vi "pharmaBot_v0.019.vi"() -> ()   [LabVIEW 2015] (continued)
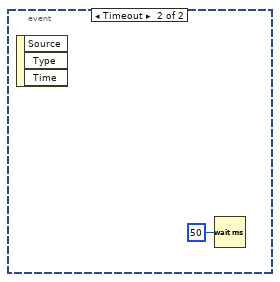
[diagram p2: hidden frame]
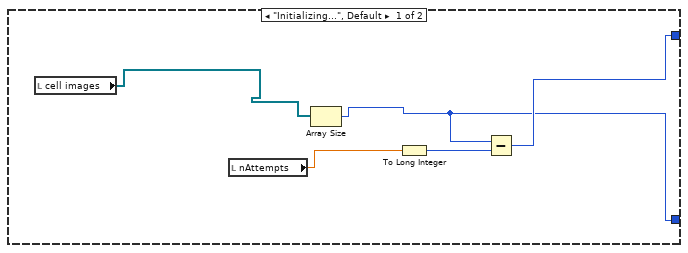
[diagram p4: hidden frame]
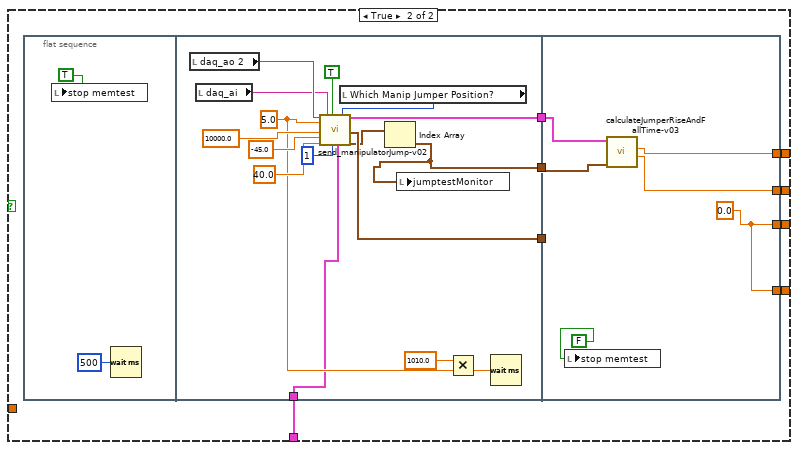
[diagram p14: hidden frame]
              }
              frame "manipulator 2" {
                n1843 = Unbundle By Name(w2697) -> ("manip 2"=w2696:refnum<vi>)
              }
              frame "manipulator 3" {
                n1844 = Unbundle By Name(w2699) -> ("manip 3"=w2698:refnum<vi>)
              }
              frame "manipulator 4" {
                n1845 = Unbundle By Name(w2701) -> ("manip 4"=w2700:refnum<vi>)
              }
            }
            n1846 = property class="Clust (strict)"(reference=w2692) -> (error out=w2689:errorcluster, "Value"=w2691:T25)  [unwired: 1 in, 1 out]
            n1847 = Unbundle By Name(w2691) -> ("actuator"=w2687:T26, "gamma (deg)"=w2678:dbl)
            n1848 = expression code="(x/180.0)*pi" "degrees to radians"(w2678) -> (w2677:dbl)
            n1849 = Unbundle By Name(w2687) -> ("Actuator COM"=w2684:refnum<visa-resource-name>)  [unwired: 1 out]
            n1850 = Sine(x=w2677) -> (sin(x)=w2675:dbl)
            n1851 = Cosine(x=w2677) -> (cos(x)=w2676:dbl)
            n1852 = call "sc_adjustMotion.vi"("error in (no error)"=w2689, "motion"=scope_motion."fast", "VISA handle"=w2684) -> ("error out"=w2688:errorcluster)  [unwired: 7 in, 1 out]
            n1853 = Multiply(x=w2674, y=w2676) -> (x*y=w2672:dbl)
            n1854 = Multiply(x=w2674, y=w2675) -> (x*y=w2673:dbl)
            n1855 = Build Array(w2672, 0, w2673) -> (w2682:dbl[])
            n1856 = call "move manipulator abs xyz.vi"("blocking?"=TRUE, "which manipulator"=w2683, "error in (no error)"=w2688, "transform cluster + actuator"=w2680, "positions"=w2681, "location (steps)"=w2682) -> ("error out"=w2685:errorcluster)  [unwired: 5 in]
            n1857 = call "sc_adjustMotion.vi"("error in (no error)"=w2685, "motion"=scope_motion."slow_dualPatch", "VISA handle"=w2684) -> ()  [unwired: 7 in, 2 out]
          }
        }
      }
      event "save locations", "save locations 2": Value Change {
        n1858 = event-data() -> ("NewVal"=w2704:bool)  [unwired: 1 in, 5 out]
        n1859 = case shown="True" w2704 {
          tunnel: w2703 -> [_ w2726]
          frame False {
          }
          frame True {
            n1860 = local read "cleaning bath loc 1"() -> (w2724:i32[])
            n1861 = local read "cleaning bath loc 2"() -> (w2721:i32[])
            n1862 = local read "loc above baths 1"() -> (w2725:i32[])
            n1863 = local read "loc above baths 2"() -> (w2722:i32[])
            n1864 = local read "wash bath loc 1"() -> (w2723:i32[])
            n1865 = local read "wash bath loc 2"() -> (w2720:i32[])
            n1866 = Wait (ms)(milliseconds to wait=u32 500) -> ()  [unwired: 1 out]
            n1867 = local read "Jumper Position o-C"() -> (w2719:dbl[])
            n1868 = local read "Jumper Position C-o"() -> (w2718:dbl[])
            n1869 = local read "Jumper Position C-B"() -> (w2717:dbl[])
            n1870 = local read "Jumper Position B-C"() -> (w2716:dbl[])
            n1871 = local read "Jumper Position B-A"() -> (w2715:dbl[])
            n1872 = local read "Jumper Position A-B"() -> (w2714:dbl[])
            n1873 = local read "Jumper Position A-o"() -> (w2713:dbl[])
            n1874 = local read "Jumper Position o-A"() -> (w2712:dbl[])
            n1875 = local read "Jumper Position C"() -> (w2711:dbl[])
            n1876 = local read "Jumper Position B"() -> (w2710:dbl[])
            n1877 = local read "Jumper Position A"() -> (w2709:dbl[])
            n1878 = local read "Experiment Safe Position"() -> (w2708:dbl[])
            n1879 = local read "Jumper Safe Position"() -> (w2707:dbl[])
            n1880 = Open/Create/Replace File(file path (use dialog)=w2726, operation (0:open)=T61."open or create") -> (refnum out=w2730:refnum<file>, cancelled=w2727:bool, error out=w2731:errorcluster)  [unwired: 4 in]
            n1881 = Build Array(w2725, w2724, w2723, w2722, w2721, w2720, w2719, w2718, w2717, w2716, w2715, w2714, w2713, w2712, w2711, w2710, w2709, w2708, w2707) -> (w2705:dbl[][])
            n1882 = Flatten To String(anything=w2705) -> (data string=w2729:string)  [unwired: 3 in, 2 out]
            n1883 = case shown="False" w2727 {
              tunnel: w2731 -> [w2737 _]
              tunnel: w2730 -> [w2736 _]
              tunnel: w2729 -> [w2735 _]
              frame False {
                n1884 = Write to Text File(file (use dialog)=w2736, text=w2735, error in=w2737) -> (refnum out=w2733:refnum<file>, error out=w2734:errorcluster)  [unwired: 1 in, 1 out]
                n1885 = Close File(refnum=w2733, error in=w2734) -> (path=w2732:path)  [unwired: 1 out]
                n1886 = local write "save path"(w2732) -> ()
              }
              frame True {
              }
            }
            n1887 = local write "mock location array"(w2705) -> ()
          }
        }
      }
      event "load HEK/slice params": Value Change {
        n1888 = event-data() -> ("NewVal"=w2753:bool)  [unwired: 1 in, 5 out]
        n1889 = control-ref of="gigasealing options"() -> (w2740:refnum<vi>)
        n1890 = control-ref of="GS timeout (s)"() -> (w2742:refnum<vi>)
        n1891 = control-ref of="vertical z dist (vertical rel only)  (px)"() -> (w2741:refnum<vi>)
        n1892 = control-ref of="NH wait time (ms)"() -> (w2739:refnum<vi>)
        n1893 = control-ref of="hunt pressure (mBar)"() -> (w2754:refnum<vi>)
        n1894 = control-ref of="holding V (mV)"() -> (w2752:refnum<vi>)
        n1895 = control-ref of="Extra threshold (MOhms)"() -> (w2751:refnum<vi>)
        n1896 = control-ref of="Neuron Detection Threshold (MOhms)"() -> (w2750:refnum<vi>)
        n1897 = control-ref of="Pipette broken threshold (MOhms)"() -> (w2749:refnum<vi>)
        n1898 = control-ref of="max hunt distance (um)"() -> (w2748:refnum<vi>)
        n1899 = control-ref of="above dist (approach above only) (steps)"() -> (w2747:refnum<vi>)
        n1900 = control-ref of="subtract from distToDescend (steps)"() -> (w2746:refnum<vi>)
        n1901 = control-ref of="NH step size (steps)"() -> (w2745:refnum<vi>)
        n1902 = control-ref of="NH method"() -> (w2744:refnum<vi>)
        n1903 = control-ref of="initial positioning"() -> (w2743:refnum<vi>)
        n1904 = case shown="True" w2753 {
          tunnel: w2754 -> [_ w2786]
          tunnel: w2752 -> [_ w2785]
          tunnel: w2751 -> [_ w2784]
          tunnel: w2750 -> [_ w2783]
          tunnel: w2749 -> [_ w2782]
          tunnel: w2748 -> [_ w2781]
          tunnel: w2747 -> [_ w2780]
          tunnel: w2746 -> [_ w2779]
          tunnel: w2745 -> [_ w2778]
          tunnel: w2744 -> [_ w2777]
          tunnel: w2743 -> [_ w2765]
          tunnel: w2742 -> [_ w2763]
          tunnel: w2741 -> [_ w2760]
          tunnel: w2740 -> [_ w2759]
          tunnel: w2739 -> [_ w2757]
          frame False {
          }
          frame True {
            # "LOADING"
            n1905 = case shown="\"slice\", Default" "HEK/slice options" {
              tunnel: ["hunt pressure (mBar) slice" "hunt pressure (mBar) slice HEK"] -> w2775
              tunnel: ["holding V (mV) slice" "holding V (mV) slice HEK"] -> w2774
              tunnel: ["Extra threshold (MOhms) slice" "Extra threshold (MOhms) slice HEK"] -> w2773
              tunnel: ["Neuron Detection Threshold (MOhms) slice" "Neuron Detection Threshold (MOhms) slice HEK"] -> w2772
              tunnel: ["Pipette broken threshold (MOhms) slice" "Pipette broken threshold (MOhms) slice HEK"] -> w2771
              tunnel: ["max hunt distance (um) slice" "max hunt distance (um) slice HEK"] -> w2770
              tunnel: ["d(above cell) (steps) (used to be 10) slice" "d(above cell) (steps) (used to be 10) slice HEK"] -> w2769
              tunnel: ["approach above cell (steps) slice" "approach above cell (steps) HEK"] -> w2768
              tunnel: ["NH step size (steps) slice" "NH step size (steps) slice HEK"] -> w2767
              tunnel: ["NH method slice" "NH method slice HEK"] -> w2766
              tunnel: [approach_type."approach above" ("Value") approach_type."vertical rel" ("Value")] -> w2764
              tunnel: ["GS timeout (s) slice" "GS timeout (s) HEK"] -> w2762
              tunnel: [w2790 "vertical z dist (vertical rel only) HEK"] -> w2761
              tunnel: w2760 -> [w2791 _]
              tunnel: ["gigasealing options slice" "gigasealing options HEK"] -> w2758
              tunnel: w2757 -> [w2787 w2805]
              tunnel: [w2787 w2805] -> w2756
              tunnel: ["NH wait time (ms) slice" "NH wait time (ms) HEK"] -> w2755
              frame "slice", Default {
                n1906 = property class="DigNum (strict)"(reference=w2791) -> ("Value"=w2790:dbl)  [unwired: 1 in, 2 out]
              }
              frame "HEK" {
              }
            }
            n1907 = property class="DigNum (strict)"(reference=w2786, "Value"=w2775) -> ()  [unwired: 1 in, 2 out]
            n1908 = property class="DigNum (strict)"(reference=w2785, "Value"=w2774) -> ()  [unwired: 1 in, 2 out]
            n1909 = property class="DigNum (strict)"(reference=w2784, "Value"=w2773) -> ()  [unwired: 1 in, 2 out]
            n1910 = property class="DigNum (strict)"(reference=w2783, "Value"=w2772) -> ()  [unwired: 1 in, 2 out]
            n1911 = property class="DigNum (strict)"(reference=w2782, "Value"=w2771) -> ()  [unwired: 1 in, 2 out]
            n1912 = property class="DigNum (strict)"(reference=w2781, "Value"=w2770) -> ()  [unwired: 1 in, 2 out]
            n1913 = property class="DigNum (strict)"(reference=w2780, "Value"=w2768) -> ()  [unwired: 1 in, 2 out]
            n1914 = property class="DigNum (strict)"(reference=w2779, "Value"=w2769) -> ()  [unwired: 1 in, 2 out]
            n1915 = property class="DigNum (strict)"(reference=w2778, "Value"=w2767) -> ()  [unwired: 1 in, 2 out]
            n1916 = property class="DigNum (strict)"(reference=w2763, "Value"=w2762) -> ()  [unwired: 1 in, 2 out]
            n1917 = property class="DigNum (strict)"(reference=w2756, "Value"=w2755) -> ()  [unwired: 1 in, 2 out]
            n1918 = property class="DigNum (strict)"(reference=w2760, "Value"=w2761) -> ()  [unwired: 1 in, 2 out]
            n1919 = property class="Enum (strict)"(reference=w2777, "Value"=w2766) -> ()  [unwired: 1 in, 2 out]
            n1920 = property class="Enum (strict)"(reference=w2765, "Value"=w2764) -> ()  [unwired: 1 in, 2 out]
            n1921 = property class="Clust (strict)"(reference=w2759, "Value"=w2758) -> ()  [unwired: 1 in, 2 out]
          }
        }
      }
      event "load Settings": Value Change {
        n1922 = event-data() -> ("NewVal"=w2821:bool)  [unwired: 1 in, 5 out]
        n1923 = local read "allMainVIcontrols"() -> (w2820:refnum<vi>[])
        n1924 = case shown="True" w2821 {
          tunnel: w2820 -> [_ w2824]
          frame False {
          }
          frame True {
            n1925 = call "load config"() -> ("selected path"=w2823:path, "cancelled"=w2822:bool)  [unwired: 12 in, 2 out]
            n1926 = case shown="False" w2822 {
              tunnel: w2824 -> [w2827 _]
              tunnel: w2823 -> [w2825 _]
              frame False {
                n1927 = call "Read and Write Controls to Automatic Config File.vi"("Action"=RWC_Actions."Read", "Control References"=w2827, "filepath"=w2825) -> ()  [unwired: 8 in, 1 out]
                "config file" <- w2825
              }
              frame True {
              }
            }
          }
        }
      }
      event "check Power Specturm": Value Change {
        n1928 = event-data() -> ("NewVal"=w2828:bool)  [unwired: 1 in, 5 out]
        n1929 = local write "stop memtest"(w2828) -> ()
      }
      event "load clean": Value Change {
        n1930 = event-data() -> ("NewVal"=w2830:bool)  [unwired: 1 in, 5 out]
        n1931 = case shown="True" w2830 {
          frame False {
          }
          frame True {
            n1932 = Open/Create/Replace File() -> (refnum out=w2831:refnum<file>, cancelled=w2833:bool, error out=w2832:errorcluster)  [unwired: 6 in]
            n1933 = case shown="False" w2833 {
              tunnel: w2832 -> [w2835 _]
              tunnel: w2831 -> [w2836 _]
              frame False {
                n1934 = Read from Text File(file (use dialog)=w2836, error in=w2835) -> (refnum out=w2839:refnum<file>, text=w2837:string)  [unwired: 2 in, 2 out]
                n1935 = Unflatten From String(type=dbl[][] [] ("appended array"), binary string=w2837) -> (value=w2834:dbl[][], error out=w2838:errorcluster)  [unwired: 3 in, 1 out]
                n1936 = local write "Cleaning step (time [s], value [mBar]) actual"(w2834) -> ()
                n1937 = Close File(refnum=w2839, error in=w2838) -> ()  [unwired: 2 out]
              }
              frame True {
              }
            }
          }
        }
      }
      event "load wash": Value Change {
        n1938 = event-data() -> ("NewVal"=w2842:bool)  [unwired: 1 in, 5 out]
        n1939 = case shown="True" w2842 {
          frame False {
          }
          frame True {
            n1940 = Open/Create/Replace File() -> (refnum out=w2844:refnum<file>, cancelled=w2845:bool, error out=w2843:errorcluster)  [unwired: 6 in]
            n1941 = case shown="False" w2845 {
              tunnel: w2844 -> [w2849 _]
              tunnel: w2843 -> [w2848 _]
              frame False {
                n1942 = Read from Text File(file (use dialog)=w2849, error in=w2848) -> (refnum out=w2847:refnum<file>, text=w2851:string, error out=w2852:errorcluster)  [unwired: 2 in, 1 out]
                n1943 = Unflatten From String(type=dbl[][] [] ("appended array"), binary string=w2851, error in (no error)=w2852) -> (value=w2846:dbl[][], error out=w2850:errorcluster)  [unwired: 2 in, 1 out]
                n1944 = local write "Wash step (time [s], value [mBar]) actual"(w2846) -> ()
                n1945 = Close File(refnum=w2847, error in=w2850) -> ()  [unwired: 2 out]
              }
              frame True {
              }
            }
          }
        }
      }
      event "set park location": Value Change {
        n1946 = event-data() -> ("NewVal"=w2855:bool)  [unwired: 1 in, 5 out]
        n1947 = case shown="True" w2855 {
          frame False {
          }
          frame True {
            n1948 = local read "current stage location (px)"() -> (w2856:dbl[])
            n1949 = Index Array(array=w2856, index=2) -> (element=w2857:dbl)
            n1950 = local write "park plane z (px)"(w2857) -> ()
          }
        }
      }
      event "Adjust exposure (ms)": Value Change {
        n1951 = event-data() -> ("NewVal"=w2860:dbl)  [unwired: 1 in, 5 out]
        n1952 = local read "cam info out"() -> (w2862:T38)
        n1953 = local read "orig image"() -> (w2861:T10)
        n1954 = call "close_cam_topLvl_v02.vi"("cam info in"=w2862) -> ("error out"=w2863:errorcluster)  [unwired: 10 in]
        n1955 = call "init_cam_topLvl_v02.vi"("error in"=w2863, "exposure (ms)"=w2860, "orig image"=w2861, "cam info in"=w2862) -> ()  [unwired: 6 in, 2 out]
      }
      event "go to cleaning bath loc", "go to wash bath loc", "go to loc above baths": Value Change {
        n1956 = event-data() -> ("NewVal"=w2867:bool)  [unwired: 1 in, 5 out]
        n1957 = case shown="True" w2867 {
          tunnel: w2866 -> [_ w2884]
          tunnel: w2865 -> [_ w2883]
          frame False {
          }
          frame True {
            # "first tab -> manip 1\nsecond tab -> manip 2\netc"
            n1958 = local read "loc above baths 1"() -> (w2870:i32[])
            n1959 = local read "loc above baths 2"() -> (w2871:i32[])
            n1960 = Equal?(x="cleaning tab", y=enum32{"manip 1", "manip 2"}."manip 1" ("cleaning tab")) -> (x = y?=w2869:bool)
            n1961 = Select(t=w2870, s=w2869, f=w2871) -> (s? t:f=w2868:i32[])
            n1962 = local read "cleaning bath loc 1"() -> (w2874:i32[])
            n1963 = local read "cleaning bath loc 2"() -> (w2873:i32[])
            n1964 = Select(t=w2868, s="go to loc above baths", f=i32[] []) -> (s? t:f=w2889:i32[])
            n1965 = Select(t=w2874, s=w2869, f=w2873) -> (s? t:f=w2872:i32[])
            n1966 = Select(t=T8."manipulator 1" ("which manipulator"), s=w2869, f=T8."manipulator 2" ("which manipulator")) -> (s? t:f=w2879:T8)
            n1967 = Select(t=w2872, s="go to cleaning bath loc", f=w2889) -> (s? t:f=w2891:i32[])
            n1968 = local read "wash bath loc 1"() -> (w2877:i32[])
            n1969 = local read "wash bath loc 2"() -> (w2876:i32[])
            n1970 = Select(t=w2877, s=w2869, f=w2876) -> (s? t:f=w2875:i32[])
            n1971 = Select(t=w2875, s="go to wash bath loc", f=w2891) -> (s? t:f=w2882:i32[])
            n1972 = call "move manipulator abs xyz.vi"("blocking?"=TRUE, "which manipulator"=w2879, "transform cluster + actuator"=w2883, "positions"=w2884, "location (steps)"=w2882) -> ()  [unwired: 6 in, 1 out]
          }
        }
      }
    }
  }
  n1973 = call "IMAQ Create"("Image Name"="cell mask", "Image Type"=w652) -> ("New Image"=w650:T10, "error out"=w624:errorcluster)  [unwired: 3 in]
  n1974 = case shown="False" w247 {
    tunnel: w701 -> [w2904 _]
    frame False {
      # "init daq to\nstart square pulse\nfor R measurement"
      n1975 = local read "daq_ai"() -> (w2893:tag)
      n1976 = local read "daq_ao"() -> (w2894:tag)
      n1977 = local read "Memtest inputs"() -> (w2901:T29)
      n1978 = call "init_memtest_1channel.vi"("memtest"=w2901, "AO physical channels"=w2894, "AI Physical Channels"=w2893) -> ("AO error out"=w2898:errorcluster, "AO task out"=w2902:refnum<k21>, "AI task out"=w2903:refnum<k21>)  [unwired: 4 in, 2 out]
      n1979 = while {
        tunnel: w2904 -> [_]
        tunnel: w2901 -> [w2910]
        tunnel: [w2912] -> w2899
        tunnel: w2898 -> [w2911]
        tunnel: [w2910] -> w2897
        shift-right: [w2913] -> w2900
        shift-left: w2903 -> [w2915]
        shift-right: [w2909] -> w2896
        shift-left: w2902 -> [w2914]
        tunnel: w2894 -> [w2908]
        tunnel: w2893 -> [w2906]
        stop <- w2905 stop-if-true
        n1980 = local read "stop memtest"() -> (w2907:bool)
        n1981 = case shown="False" w2907 {
          tunnel: w2915 -> [w2936 w2945]
          tunnel: w2914 -> [w2935 w2944]
          tunnel: [w2934 w2942] -> w2913
          tunnel: [w2933 w2940] -> w2912
          tunnel: w2911 -> [w2932 w2943]
          tunnel: w2910 -> [w2931 w2939]
          tunnel: [w2930 w2941] -> w2909
          tunnel: w2908 -> [_ w2946]
          tunnel: w2906 -> [_ w2937]
          frame False {
            # "read resistance"
            n1982 = call "advanced_cont_memtest_1channel-v06.vi"("Pulse AI task in"=w2936, "replicates"=5, "Pulse AO task in"=w2935, "error in"=w2932, "memtest"=w2931, "which clamp"=enum16{"VClamp", "IClamp"}."VClamp") -> ("avg peak height"=w2919:dbl, "Pulse AI task out"=w2934:refnum<k21>, "data out (pA or mV)"=w2918:waveform(dbl)[], "cell stats"=w2920:T5, "Pulse AO task out"=w2930:refnum<k21>, "error out"=w2933:errorcluster)  [unwired: 5 in, 3 out]
            n1983 = local write "cell stats"(w2920) -> ()
            n1984 = Unbundle By Name(w2920) -> ("Rt (MOhms)"=w2928:dbl, "Ihold (pA)"=w2927:dbl, "Cm (pF)"=w2926:dbl, "Ra (MOhms)"=w2925:dbl)
            n1985 = Unbundle By Name(w2920) -> ("Rt (MOhms)"=w2924:dbl, "Ihold (pA)"=w2923:dbl, "Cm (pF)"=w2922:dbl, "Ra (MOhms)"=w2921:dbl)
            n1986 = Index Array(array=w2918) -> (element=w2917:waveform(dbl))  [unwired: 1 in]
            n1987 = local write "P1"(w2924) -> ()
            n1988 = local write "P2"(w2928) -> ()
            n1989 = local write "Iholding 2"(w2927) -> ()
            n1990 = local write "Iholding 1"(w2923) -> ()
            n1991 = local write "Cm 2"(w2926) -> ()
            n1992 = local write "Ra 2"(w2925) -> ()
            n1993 = local write "Ra 1"(w2921) -> ()
            n1994 = local write "Cm 1"(w2922) -> ()
            n1995 = local write "memtest 1"(w2917) -> ()
            n1996 = local write "avg peak height 1"(w2919) -> ()
            n1997 = local write "avg peak height 2"(w2919) -> ()
          }
          frame True {
            n1998 = local read "check Power Specturm"() -> (w2938:bool)
            n1999 = case shown="True" w2938 {
              tunnel: w2946 -> [w2949 w2995]
              tunnel: w2945 -> [w2966 w2994]
              tunnel: w2944 -> [w2965 w2993]
              tunnel: w2943 -> [w2964 w2992]
              tunnel: [w2962 w2990] -> w2942
              tunnel: [w2961 w2989] -> w2941
              tunnel: [w2960 w2988] -> w2940
              tunnel: w2939 -> [w2954 w2987]
              tunnel: w2937 -> [w2955 _]
              frame True {
                # "stops memtest"
                # "loops while WC program is running"
                n2000 = local read "Power Spectrum inputs"() -> (w2947:T29)
                n2001 = call "close_memtest_N_v02.vi"("which clamp"=enum16{"VClamp", "IClamp"}."VClamp", "memtest"=w2954, "AO physical channels"=w2949, "AI error in"=w2964, "AO task in"=w2965, "AI task in"=w2966) -> ("error out"=w2959:errorcluster)  [unwired: 5 in]
                n2002 = call "init_memtest_1channel_justNoise_v02.vi"("memtest"=w2947, "AO error in"=w2959, "AO physical channels"=w2949, "AI Physical Channels"=w2955) -> ("AO error out"=w2958:errorcluster, "AO task out"=w2956:refnum<k21>, "AI task out"=w2957:refnum<k21>)  [unwired: 3 in, 2 out]
                n2003 = while {
                  tunnel: w2958 -> [w2982]
                  tunnel: [w2981] -> w2953
                  shift-right: [w2976] -> w2950
                  shift-left: w2957 -> [w2979]
                  shift-right: [w2975] -> w2951
                  shift-left: w2956 -> [w2978]
                  tunnel: w2947 -> [w2980]
                  tunnel: [w2974] -> w2948
                  stop <- w2972 continue-if-true
                  w2974 = enum16{"VClamp", "IClamp"}."VClamp" ("which clamp")
                  n2004 = call "advanced_cont_memtest_1channel-v05justNoise.vi"("Pulse AI task in"=w2979, "replicates"=5, "Pulse AO task in"=w2978, "error in"=w2982, "memtest"=w2980, "which clamp"=w2974) -> ("Power Spectrum"=w2977:dbl[], "Pulse AI task out"=w2976:refnum<k21>, "data out (pA or mV)"=w2969:waveform(dbl)[], "cell stats"=w2984:T5, "Pulse AO task out"=w2975:refnum<k21>, "error out"=w2981:errorcluster)  [unwired: 6 in, 2 out]
                  n2005 = local write "cell stats"(w2984) -> ()
                  n2006 = local write "Power Spectrum"(w2977) -> ()
                  n2007 = Index Array(array=w2969) -> (element=w2973:waveform(dbl))  [unwired: 1 in]
                  n2008 = local write "Power Spectrum Current"(w2969) -> ()
                  n2009 = local read "check Power Specturm"() -> (w2985:bool)
                  n2010 = local write "memtest 1"(w2973) -> ()
                  n2011 = local read "stop always"() -> (w2971:bool)
                  n2012 = Not(x=w2971) -> (.not. x?=w2970:bool)
                  n2013 = And(x=w2970, y=w2985) -> (x .and. y?=w2972:bool)
                  n2014 = Wait (ms)(milliseconds to wait=u32 200) -> ()  [unwired: 1 out]
                }
                n2015 = call "close_memtest_N_v02.vi"("which clamp"=w2948, "memtest"=w2947, "AO physical channels"=w2949, "AI error in"=w2953, "AO task in"=w2951, "AI task in"=w2950) -> ("error out"=w2952:errorcluster)  [unwired: 5 in]
                n2016 = local read "daq_ai"() -> (w2968:tag)
                n2017 = local read "daq_ao"() -> (w2967:tag)
                n2018 = call "init_memtest_1channel.vi"("memtest"=w2954, "AO error in"=w2952, "AO physical channels"=w2967, "AI Physical Channels"=w2968) -> ("AO error out"=w2960:errorcluster, "AO task out"=w2961:refnum<k21>, "AI task out"=w2962:refnum<k21>)  [unwired: 3 in, 2 out]
              }
              frame False {
                # "stops memtest"
                # "loops while WC program is running"
                n2019 = call "close_memtest_N_v02.vi"("which clamp"=enum16{"VClamp", "IClamp"}."VClamp", "memtest"=w2987, "AO physical channels"=w2995, "AI error in"=w2992, "AO task in"=w2993, "AI task in"=w2994) -> ("error out"=w2997:errorcluster)  [unwired: 5 in]
                n2020 = while {
                  tunnel: w2997 -> [w3002]
                  tunnel: [w3002] -> w2996
                  stop <- w3001 continue-if-true
                  n2021 = local read "stop memtest"() -> (w3001:bool)
                  n2022 = Wait (ms)(milliseconds to wait=u32 200) -> ()  [unwired: 1 out]
                }
                n2023 = local read "daq_ai"() -> (w2999:tag)
                n2024 = local read "daq_ao"() -> (w2998:tag)
                n2025 = call "init_memtest_1channel.vi"("memtest"=w2987, "AO error in"=w2996, "AO physical channels"=w2998, "AI Physical Channels"=w2999) -> ("AO error out"=w2988:errorcluster, "AO task out"=w2989:refnum<k21>, "AI task out"=w2990:refnum<k21>)  [unwired: 3 in, 2 out]
              }
            }
          }
        }
        n2026 = local read "stop always"() -> (w2905:bool)
      }
      n2027 = call "close_memtest_N_v02.vi"("which clamp"=enum16{"VClamp", "IClamp"}."VClamp", "memtest"=w2897, "AO physical channels"=w2894, "AI error in"=w2899, "AO task in"=w2896, "AI task in"=w2900) -> ()  [unwired: 5 in, 1 out]
    }
    frame True {
      n2028 = while {
        stop <- w3007 stop-if-true
        n2029 = local read "pipette 2 I (pA)"() -> (w3006:dbl)
        n2030 = local read "demo pipette 2 R (MOhms)"() -> (w3005:dbl)
        n2031 = local read "pipette 1 I (pA)"() -> (w3004:dbl)
        n2032 = local read "demo pipette 1 R (MOhms)"() -> (w3003:dbl)
        n2033 = local write "Iholding 2"(w3006) -> ()
        n2034 = local write "Iholding 1"(w3004) -> ()
        n2035 = local write "P2"(w3005) -> ()
        n2036 = local write "P1"(w3003) -> ()
        n2037 = local read "stop always"() -> (w3007:bool)
      }
    }
  }
  n2038 = local read "daq_do 2"() -> (w259:tag)
  n2039 = case shown="True" w284 {
    tunnel: w259 -> [_ w3008]
    frame False {
    }
    frame True {
      n2040 = while {
        tunnel: w3008 -> [w3013]
        stop <- w3014 stop-if-true
        n2041 = local read "Valve2 Go"() -> (w3012:bool)
        n2042 = local read "V2-Changing"() -> (w3011:bool)
        n2043 = Or(x=w3012, y=w3011) -> (x .or. y?=w3010:bool)
        n2044 = case shown="True" w3010 {
          tunnel: w3013 -> [_ w3019]
          frame False {
          }
          frame True {
            n2045 = local read "V2-State"() -> (w3018:u16)
            n2046 = local read "Valve2"() -> (w3017:u16)
            n2047 = Not Equal?(x=w3017, y=w3018) -> (x != y?=w3015:bool)
            n2048 = case shown="True" w3015 {
              tunnel: w3017 -> [_ w3025]
              tunnel: w3019 -> [_ w3024]
              tunnel: [w3020 w3023] -> w3016
              tunnel: w3018 -> [w3020 w3022]
              frame False {
              }
              frame True {
                n2049 = call "sendValveSignal-v05.vi"("daq_do"=w3024, "ChangeToValve"=w3025, "CurrentValve"=w3022, "Set Status"=FALSE) -> ("ValveSetTo"=w3023:u16)  [unwired: 4 in, 2 out]
              }
            }
            n2050 = local write "V2-Changing"(w3015) -> ()
            n2051 = local write "V2-State"(w3016) -> ()
          }
        }
        n2052 = Wait (ms)(milliseconds to wait=u32 100) -> ()  [unwired: 1 out]
        n2053 = local read "stop always"() -> (w3014:bool)
      }
    }
  }
  n2054 = property on="tracking" class="Bool (strict)"(error in=w624, "Value"=w625) -> (error out=w626:errorcluster)  [unwired: 1 in, 1 out]
  n2055 = local read "daq_do 1"() -> (w258:tag)
  n2056 = case shown="True" w287 {
    tunnel: w258 -> [_ w3026]
    frame False {
    }
    frame True {
      n2057 = while {
        tunnel: w3026 -> [w3031]
        stop <- w3032 stop-if-true
        n2058 = local read "Valve1 Go"() -> (w3030:bool)
        n2059 = local read "V1-Changing"() -> (w3029:bool)
        n2060 = Or(x=w3030, y=w3029) -> (x .or. y?=w3028:bool)
        n2061 = case shown="True" w3028 {
          tunnel: w3031 -> [_ w3037]
          frame False {
          }
          frame True {
            n2062 = local read "V1-State"() -> (w3036:u16)
            n2063 = local read "Valve1"() -> (w3035:u16)
            n2064 = Not Equal?(x=w3035, y=w3036) -> (x != y?=w3033:bool)
            n2065 = case shown="True" w3033 {
              tunnel: w3035 -> [_ w3043]
              tunnel: w3037 -> [_ w3042]
              tunnel: [w3038 w3041] -> w3034
              tunnel: w3036 -> [w3038 w3040]
              frame False {
              }
              frame True {
                n2066 = call "sendValveSignal-v05.vi"("daq_do"=w3042, "ChangeToValve"=w3043, "CurrentValve"=w3040, "Set Status"=FALSE) -> ("ValveSetTo"=w3041:u16)  [unwired: 4 in, 2 out]
              }
            }
            n2067 = local write "V1-Changing"(w3033) -> ()
            n2068 = local write "V1-State"(w3034) -> ()
          }
        }
        n2069 = Wait (ms)(milliseconds to wait=u32 100) -> ()  [unwired: 1 out]
        n2070 = local read "stop always"() -> (w3032:bool)
      }
    }
  }
  n2071 = call "IMAQ Create"("Image Name"="deconv output", "Image Type"=w648) -> ("New Image"=w647:T10, "error out"=w646:errorcluster)  [unwired: 3 in]
  n2072 = property on="init tracker success" class="Bool (strict)"(error in=w626, "Value"=w625) -> (error out=w623:errorcluster)  [unwired: 1 in, 1 out]
  n2073 = while {
    tunnel: w623 -> [w3051]
    tunnel: w650 -> [w3050]
    tunnel: w647 -> [w3049]
    tunnel: w646 -> [w3048]
    shift-right: [w3044] -> _
    shift-left: w453 -> [w3047]
    shift-right: [w3045] -> _
    shift-left: w453 -> [w3046]
    stop <- w3052 stop-if-true
    n2074 = local read "tracking"() -> (w3053:bool)
    n2075 = case shown="True" w3053 {
      tunnel: w3051 -> [_ w3087]
      tunnel: w3050 -> [_ w3086]
      tunnel: w3049 -> [_ w3081]
      tunnel: w3048 -> [_ w3080]
      tunnel: w3046 -> [_ w3070]
      tunnel: w3047 -> [_ w3076]
      tunnel: [w3054 w3068] -> w3045
      tunnel: [w3054 w3055] -> w3044
      frame False {
        w3054 = dbl[][] []
      }
      frame True {
        # "for john's pipette blanking algorithm\nfeed in X Y pixel location of pipette and\nZ location of pipette-stage (so it is normalized)"
        # "this should be manip dependent!!!"
        # "if cell tracking is good\n-> update centroid\n\nelse\n-> do not update"
        n2076 = local read "pipette_px_onscreen"() -> (w3065:dbl[])
        n2077 = local read "Slice view"() -> (w3089:T10)
        n2078 = call "IMAQ ImageToArray"("Image"=w3089) -> ("Image Pixels (U8)"=w3084:u8[][])  [unwired: 3 in, 4 out]
        n2079 = script code="% run tracking script\nrun_cellTracker_flag = 0;\nrun_cellTracker;\n\n% 2/18/17 find centroid\nlogical_mask = logical(cell_mask);\nstat = regionprops(logical_mask, 'centroid');\n\n% 4/8/17 if not found, centroid is screen center\nif isempty(stat)\n    centroid_px = [size(LV_image,2) size(LV_image,1)]/2;\nelse\n    centroid_px = stat.Centroid;\nend\n\n% 4/10/17\npipette_px = pipette_coords\ncell_detected = Features.cell_detected;\npipette_detected = Features.pipette_detected;\npipette_correlation = Features.pipette_corr_pwr;"("LV_image"=w3084, "pipette_px_onscreen"=w3065) -> ("??"=w3064:errorcluster, "cell_mask"=w3088:dbl[][], "run_cellTracker_flag"=w3085:dbl, "deconv_output"=w3082:dbl[][], "centroid_px"=w3078:dbl[], "cell_detected"=w3061:dbl, "pipette_detected"=w3062:dbl, "pipette_correlation"=w3063:dbl)  [unwired: 1 in, 1 out]
        n2080 = local read "current pipette locations (px)"() -> (w3067:dbl[][])
        n2081 = Not Equal To 0?(x=w3085) -> (x != 0?=w3058:bool)
        n2082 = Index Array(array=w3067, index (row)=0) -> (element=w3057:dbl[])  [unwired: 1 in]
        n2083 = Build Array (concatenate)(w3078, 0.0) -> (w3069:dbl[])
        n2084 = local write "pipette_corr_pwr"(w3063) -> ()
        n2085 = call "IMAQ ArrayToImage"("error in (no error)"=w3080, "Image Pixels (U8)"=w3082, "Image"=w3081) -> ("Image Out"=w3060:T10)  [unwired: 7 in, 1 out]
        n2086 = call "IMAQ ArrayToImage"("error in (no error)"=w3087, "Image Pixels (U8)"=w3088, "Image"=w3086) -> ("error out"=w3079:errorcluster, "Image Out"=w3083:T10)  [unwired: 7 in]
        n2087 = local write "deconvolution output"(w3060) -> ()
        n2088 = local write "run tracker success"(w3058) -> ()
        n2089 = call "IMAQ MaskToROI"("Image"=w3083, "error in (no error)"=w3079) -> ("ROI Descriptor"=w3059:T28)  [unwired: 5 in, 2 out]
        n2090 = Greater Than 0?(x=w3061) -> (x > 0?=w3071:bool)
        n2091 = Build Array (concatenate)(w3076, w3057) -> (w3055:dbl[][])
        n2092 = local write "cell track error out"(w3064) -> ()
        n2093 = local write "cell mask ROI"(w3059) -> ()
        n2094 = local write "pipette_px_onscreen"(w3057) -> ()
        n2095 = case shown="True" w3071 {
          tunnel: w3069 -> [_ w3106]
          tunnel: w3070 -> [w3090 w3095]
          tunnel: w3069 -> [_ w3094]
          tunnel: [w3090 w3093] -> w3068
          frame False {
          }
          frame True {
            w3105 = 5
            n2096 = Build Array (concatenate)(w3095, w3094) -> (w3093:dbl[][])
            n2097 = Index Array(array=w3093, index (col) #1=0 ("index (row)"), index (col) #2=1 ("index (row)")) -> (element #1=w3096:dbl[], element #2=w3097:dbl[])  [unwired: 2 in]
            n2098 = Index Array(array=w3106) -> (element #1=w3104:dbl, element #2=w3103:dbl, element #3=w3100:dbl)  [unwired: 3 in]
            n2099 = Bundle(w3096, w3097) -> (w3092:cluster{dbl[], dbl[]})  [unwired: 1 in]
            n2100 = local write "cell centroid array"(w3093) -> ()
            n2101 = call <vilib>:"Mean PtByPt.vi"("x"=w3104, "sample length"=w3105) -> ("mean"=w3102:dbl)  [unwired: 2 in, 1 out]
            n2102 = call <vilib>:"Mean PtByPt.vi"("x"=w3103, "sample length"=w3105) -> ("mean"=w3101:dbl)  [unwired: 2 in, 1 out]
            n2103 = local write "cell centroid graph"(w3092) -> ()
            n2104 = Build Array(w3102, w3101, w3100) -> (w3091:dbl[])
            n2105 = local write "centroid_px"(w3091) -> ()
          }
        }
        n2106 = Index Array(array=w3055, index (col) #1=0 ("disabled index (col)"), index (col) #2=1 ("index (col)")) -> (element #1=w3074:dbl[], element #2=w3075:dbl[])  [unwired: 2 in]
        n2107 = Bundle(w3074, w3075) -> (w3056:cluster{dbl[], dbl[]})  [unwired: 1 in]
        n2108 = local write "pipette centroid graph"(w3056) -> ()
        n2109 = local write "cell_tracking_quality"(w3061) -> ()
        n2110 = local write "pipette_tracking_quality"(w3062) -> ()
        n2111 = local write "pipette centroid array"(w3055) -> ()
      }
    }
    n2112 = local read "stop always"() -> (w3052:bool)
  }
  n2113 = while {
    stop <- w3109 stop-if-true
    n2114 = event shown="[0] \"Choose Position\": Value Change" {
      selector: _ -> [_ _]
      dyn-events: _ -> [_ _]
      timeout: 50 -> [_ _]
      event "Choose Position": Value Change {
        n2115 = event-data() -> ()  [unwired: 1 in, 6 out]
        n2116 = local read "Jump o-C Good?"() -> (w3110:bool)
        n2117 = local read "Jump C-o Good?"() -> (w3111:bool)
        n2118 = local read "Jump C-B Good?"() -> (w3112:bool)
        n2119 = local read "Jump B-C Good?"() -> (w3113:bool)
        n2120 = local read "Jump B-A Good?"() -> (w3114:bool)
        n2121 = local read "Jump A-B Good?"() -> (w3115:bool)
        n2122 = local read "Jump A-o Good?"() -> (w3116:bool)
        n2123 = local read "Jump o-A Good?"() -> (w3117:bool)
        n2124 = local read "Jump Pos o-C"() -> (w3118:bool)
        n2125 = local read "Jump Pos C-o"() -> (w3119:bool)
        n2126 = local read "Jump Pos C-B"() -> (w3120:bool)
        n2127 = local read "Jump Pos B-A"() -> (w3121:bool)
        n2128 = local read "Jump Pos A-B"() -> (w3122:bool)
        n2129 = local read "Jump Pos A-o"() -> (w3123:bool)
        n2130 = local read "Jump Pos o-A"() -> (w3124:bool)
        n2131 = local read "Pos A"() -> (w3127:bool)
        n2132 = local read "Jump Pos B-C"() -> (w3125:bool)
        n2133 = local read "Pos C"() -> (w3126:bool)
        n2134 = local read "Pos B"() -> (w3128:bool)
        n2135 = local read "Experiment Safe"() -> (w3129:bool)
        n2136 = local read "Jumper Safe"() -> (w3130:bool)
        n2137 = local write "Position o-C Jump Good?"(w3110) -> ()
        n2138 = local write "Position C-o Jump Good?"(w3111) -> ()
        n2139 = local write "Position B-C Jump Good?"(w3113) -> ()
        n2140 = local write "Position B-A Jump Good?"(w3114) -> ()
        n2141 = local write "Position A-B Jump Good?"(w3115) -> ()
        n2142 = local write "Position A-o Jump Good?"(w3116) -> ()
        n2143 = local write "Position o-A Jump Good?"(w3117) -> ()
        n2144 = local write "Position C-B Jump Good?"(w3112) -> ()
        n2145 = local write "Experiment Safe Position Set"(w3129) -> ()
        n2146 = local write "Jumper Position o-C Set"(w3118) -> ()
        n2147 = local write "Jumper Position C-B Set"(w3120) -> ()
        n2148 = local write "Jumper Position B-C Set"(w3125) -> ()
        n2149 = local write "Jumper Position B-A Set"(w3121) -> ()
        n2150 = local write "Jumper Position A-B Set"(w3122) -> ()
        n2151 = local write "Jumper Position A-o Set"(w3123) -> ()
        n2152 = local write "Jumper Position o-A Set"(w3124) -> ()
        n2153 = local write "Jumper Position C Set"(w3126) -> ()
        n2154 = local write "Jumper Position B Set"(w3128) -> ()
        n2155 = local write "Jumper Position C-o Set"(w3119) -> ()
        n2156 = local write "Jumper Position A Set"(w3127) -> ()
        n2157 = local write "Jumper Safe Position Set"(w3130) -> ()
      }
      event Timeout {
        n2158 = event-data() -> ()  [unwired: 1 in, 3 out]
        n2159 = Wait (ms)(milliseconds to wait=u32 50) -> ()  [unwired: 1 out]
      }
    }
    n2160 = Wait (ms)(milliseconds to wait=u32 50) -> ()  [unwired: 1 out]
    n2161 = local read "stop always"() -> (w3109:bool)
  }
  n2162 = Close Reference(reference=w663) -> ()  [unwired: 1 in, 1 out]
  n2163 = while {
    tunnel: w322 -> [w3146]
    tunnel: w245 -> [w3145]
    stop <- w3144 stop-if-true
    n2164 = local read "P1 state"() -> (w3142:T11)
    n2165 = case shown="\"Click OK to start patcherBot!\", \"Human Positioning...\", \"In Process Calibration\"" w3142 {
      tunnel: w3146 -> [_ w3179]
      tunnel: w3145 -> [_ w3178]
      tunnel: [w3152 w3177] -> w3140
      tunnel: [w3151 w3176] -> w3139
      tunnel: [_ w3175] -> w3138
      tunnel: [_ w3174] -> w3137
      tunnel: [_ w3173] -> w3136
      tunnel: [_ w3172] -> w3135
      frame "Initializing...", Default {
        n2166 = local read "cell images"() -> (w3149:T10[])
        n2167 = local read "nAttempts"() -> (w3150:dbl)
        n2168 = Array Size(array=w3149) -> (size(s)=w3151:i32)
        n2169 = To Long Integer(number=w3150) -> (32bit integer=w3148:i32)
        n2170 = Subtract(x=w3151, y=w3148) -> (x-y=w3152:i32)
      }
      frame "Click OK to start patcherBot!", "Human Positioning...", "In Process Calibration" {
        w3170 = T8."manipulator 1" ("which manipulator")
        n2171 = local read "Jumper Filter Freq (Hz)"() -> (w3158:dbl)
        n2172 = local read "Manip Jump"() -> (w3159:bool)
        n2173 = local read "Jump Trigger"() -> (w3171:bool)
        n2174 = case shown="True" w3171 {
          tunnel: w3159 -> [_ w3214]
          tunnel: w3178 -> [_ w3213]
          tunnel: [_ w3212] -> w3175
          tunnel: [_ w3211] -> w3174
          tunnel: [_ w3210] -> w3173
          tunnel: [_ w3209] -> w3172
          tunnel: w3158 -> [_ w3208]
          frame False {
          }
          frame True {
            n2175 = case shown="False" w3214 {
              tunnel: [w3219 w3250] -> w3212
              tunnel: [w3218 w3249] -> w3211
              tunnel: [w3217 w3248] -> w3210
              tunnel: [w3216 w3247] -> w3209
              tunnel: w3213 -> [_ w3246]
              tunnel: w3208 -> [w3215 _]
              frame False {
                n2176 = flat-sequence {
                  tunnel: [w3230] -> w3222
                  tunnel: [w3227] -> w3221
                  tunnel: [w3229] -> w3220
                  tunnel: w3215 -> [w3225]
                  tunnel: w3222 -> [w3243]
                  tunnel: w3221 -> [w3244]
                  tunnel: w3220 -> [w3242]
                  tunnel: [w3241] -> w3219
                  tunnel: [w3240] -> w3218
                  tunnel: [w3239] -> w3217
                  tunnel: [w3238] -> w3216
                  frame #0 {
                    n2177 = local write "stop memtest"(TRUE ("stop memtest")) -> ()
                    n2178 = Wait (ms)(milliseconds to wait=u32 500) -> ()  [unwired: 1 out]
                  }
                  frame #1 {
                    n2179 = local read "daq_ao 2"() -> (w3237:tag)
                    n2180 = local read "daq_ai"() -> (w3232:tag)
                    n2181 = local read "Jump Polarity"() -> (w3226:bool)
                    n2182 = call "send_burleighJump-v02.vi"("daq_ao 2"=w3237, "daq_ai"=w3232, "Jump Polarity"=w3226, "Duration (s)"=1.0, "Sample Freq (Hz)"=10000.0, "Phase"=-45.0 ("Jump Delay (s)"), "Duty Cycle"=40.0 ("Jump Duration (s)"), "Jump Filter Freq (Hz)"=w3225) -> ("output cluster"=w3230:T63, "output waveform"=w3229:waveform(dbl), "protocol response"=w3228:waveform(dbl)[])  [unwired: 4 in, 1 out]
                    n2183 = Index Array(array=w3228) -> (element=w3227:waveform(dbl))  [unwired: 1 in]
                    n2184 = local write "jumptestMonitor"(w3227) -> ()
                    n2185 = Wait (ms)(milliseconds to wait=u32 1200) -> ()  [unwired: 1 out]
                  }
                  frame #2 {
                    n2186 = local write "stop memtest"(FALSE ("stop memtest")) -> ()
                    n2187 = call "calculateJumperRiseAndFallTime-v03.vi"("jumptestMonitor"=w3244, "output cluster"=w3243) -> ("fall time (ms)"=w3240:dbl, "rise time (ms)"=w3241:dbl)  [unwired: 8 in]
                    n2188 = call "calculateJumperRiseAndFallTime-v03.vi"("jumptestMonitor"=w3242, "output cluster"=w3243) -> ("fall time (ms)"=w3238:dbl, "rise time (ms)"=w3239:dbl)  [unwired: 8 in]
                  }
                }
              }
              frame True {
                n2189 = flat-sequence {
                  tunnel: [w3266] -> w3253
                  tunnel: [w3263] -> w3252
                  tunnel: [w3265] -> w3251
                  tunnel: w3246 -> [w3256]
                  tunnel: w3253 -> [w3275]
                  tunnel: w3252 -> [w3276]
                  tunnel: w3251 -> [_]
                  tunnel: [w3274] -> w3250
                  tunnel: [w3273] -> w3249
                  tunnel: [w3272] -> w3248
                  tunnel: [w3272] -> w3247
                  frame #0 {
                    n2190 = local write "stop memtest"(TRUE ("stop memtest")) -> ()
                    n2191 = Wait (ms)(milliseconds to wait=u32 500) -> ()  [unwired: 1 out]
                  }
                  frame #1 {
                    w3262 = 5.0 ("Duration (s)")
                    n2192 = local read "daq_ao 2"() -> (w3271:tag)
                    n2193 = local read "daq_ai"() -> (w3267:tag)
                    n2194 = local read "Which Manip Jumper Position?"() -> (w3259:T9)
                    n2195 = call "send_manipulatorJump-v02.vi"("daq_ao 2"=w3271, "Duration (s)"=w3262, "Sample Freq (Hz)"=10000.0, "Phase"=-45.0 ("Jump Delay (s)"), "Duty Cycle"=40.0 ("Jump Duration (s)"), "daq_ai"=w3267, "Use Current Position for Start Pos?"=TRUE, "Number of Replicates"=i16 1, "common cluster"=w3256, "Jump Position"=w3259) -> ("output cluster"=w3266:T63, "protcol waveform"=w3265:waveform(dbl), "protcol response"=w3264:waveform(dbl)[])  [unwired: 5 in, 2 out]
                    n2196 = Index Array(array=w3264) -> (element=w3263:waveform(dbl))  [unwired: 1 in]
                    n2197 = local write "jumptestMonitor"(w3263) -> ()
                    n2198 = Multiply(x=1010.0, y=w3262) -> (x*y=w3261:dbl)
                    n2199 = Wait (ms)(milliseconds to wait=w3261) -> ()  [unwired: 1 out]
                  }
                  frame #2 {
                    w3272 = 0.0 ("fall time (ms)")
                    n2200 = local write "stop memtest"(FALSE ("stop memtest")) -> ()
                    n2201 = call "calculateJumperRiseAndFallTime-v03.vi"("jumptestMonitor"=w3276, "output cluster"=w3275) -> ("fall time (ms)"=w3273:dbl, "rise time (ms)"=w3274:dbl)  [unwired: 8 in]
                  }
                }
              }
            }
          }
        }
        n2202 = local read "cell images"() -> (w3157:T10[])
        n2203 = local read "nAttempts"() -> (w3160:dbl)
        n2204 = Array Size(array=w3157) -> (size(s)=w3176:i32)
        n2205 = To Long Integer(number=w3160) -> (32bit integer=w3156:i32)
        n2206 = Decrement(x=w3156) -> (x-1=w3155:i32)
        n2207 = Greater Or Equal?(x=w3155, y=0) -> (x >= y?=w3153:bool)
        n2208 = case shown="True" w3153 {
          tunnel: w3155 -> [_ w3182]
          tunnel: w3157 -> [_ w3181]
          frame False {
          }
          frame True {
            n2209 = Index Array(array=w3181, index=w3182) -> (element=w3180:T10)
            n2210 = local write "current cell image"(w3180) -> ()
          }
        }
        n2211 = Subtract(x=w3176, y=w3156) -> (x-y=w3177:i32)
        n2212 = local read "0 mV"() -> (w3162:bool)
        n2213 = local read "-60 mV"() -> (w3163:bool)
        n2214 = local read "+40 mV"() -> (w3164:bool)
        n2215 = local read "0 mbar"() -> (w3166:bool)
        n2216 = local read "+20 mbar"() -> (w3167:bool)
        n2217 = local read "+100 mbar"() -> (w3168:bool)
        n2218 = local read "-200 mbar"() -> (w3165:bool)
        n2219 = local read "Multiclamp Handle"() -> (w3161:u32)
        n2220 = case shown="True" w3164 {
          tunnel: w3161 -> [_ w3190]
          frame False {
          }
          frame True {
            n2221 = call "mclamp_set_holding.vi"("set holding (mV)"=40.0, "Error in"=0, "Multiclamp Handle Out"=w3190) -> ()  [unwired: 7 in, 2 out]
          }
        }
        n2222 = case shown="True" w3163 {
          tunnel: w3161 -> [_ w3187]
          frame False {
          }
          frame True {
            n2223 = call "mclamp_set_holding.vi"("set holding (mV)"=-60.0, "Error in"=0, "Multiclamp Handle Out"=w3187) -> ()  [unwired: 7 in, 2 out]
          }
        }
        n2224 = control-ref of="Command pressure (mBar) 1"() -> (w3169:refnum<vi>)
        n2225 = case shown="True" w3168 {
          tunnel: w3179 -> [_ w3206]
          tunnel: w3170 -> [_ w3205]
          tunnel: w3169 -> [_ w3204]
          frame False {
          }
          frame True {
            n2226 = call "setPressure_topLvl.vi"("which manipulator"=w3205, "Slide Refnum"=w3204, "set pressure (mBar)"=100.0, "Pressure box control in"=w3206) -> ()  [unwired: 6 in, 2 out]
          }
        }
        n2227 = case shown="True" w3167 {
          tunnel: w3179 -> [_ w3202]
          tunnel: w3170 -> [_ w3201]
          tunnel: w3169 -> [_ w3200]
          frame False {
          }
          frame True {
            n2228 = call "setPressure_topLvl.vi"("which manipulator"=w3201, "Slide Refnum"=w3200, "set pressure (mBar)"=20.0, "Pressure box control in"=w3202) -> ()  [unwired: 6 in, 2 out]
          }
        }
        n2229 = case shown="True" w3162 {
          tunnel: w3161 -> [_ w3184]
          frame False {
          }
          frame True {
            n2230 = call "mclamp_set_holding.vi"("set holding (mV)"=0.0, "Error in"=0, "Multiclamp Handle Out"=w3184) -> ()  [unwired: 7 in, 2 out]
          }
        }
        n2231 = case shown="True" w3166 {
          tunnel: w3179 -> [_ w3198]
          tunnel: w3170 -> [_ w3197]
          tunnel: w3169 -> [_ w3196]
          frame False {
          }
          frame True {
            n2232 = call "setPressure_topLvl.vi"("which manipulator"=w3197, "Slide Refnum"=w3196, "set pressure (mBar)"=0.0, "Pressure box control in"=w3198) -> ()  [unwired: 6 in, 2 out]
          }
        }
        n2233 = case shown="True" w3165 {
          tunnel: w3179 -> [_ w3194]
          tunnel: w3170 -> [_ w3193]
          tunnel: w3169 -> [_ w3192]
          frame False {
          }
          frame True {
            n2234 = call "setPressure_topLvl.vi"("which manipulator"=w3193, "Slide Refnum"=w3192, "set pressure (mBar)"=-200.0, "Pressure box control in"=w3194) -> ()  [unwired: 6 in, 2 out]
          }
        }
      }
    }
    n2235 = case shown="\"Click OK to start patcherBot!\", \"Human Positioning...\", \"In Process Calibration\"" w3142 {
      tunnel: [_ w3288] -> w3133
      tunnel: [_ w3287] -> w3134
      tunnel: [_ w3286] -> w3132
      frame "Initializing...", Default {
      }
      frame "Click OK to start patcherBot!", "Human Positioning...", "In Process Calibration" {
        n2236 = local read "Which Validation Phase?"() -> (w3278:u16)
        n2237 = local read "ValidationOutputCluster"() -> (w3282:T2)
        n2238 = local read "check Validation?"() -> (w3279:bool)
        n2239 = Index Array(array=w3282, index=w3278) -> (element=w3285:T63)
        n2240 = Unbundle By Name(w3285) -> ("Number of Replicates"=w3283:i16)
        n2241 = Not Equal?(x=w3283, y=i16 0) -> (x != y?=w3281:bool)
        n2242 = And(x=w3281, y=w3279) -> (x .and. y?=w3280:bool)
        n2243 = case shown="True" w3280 {
          tunnel: w3285 -> [_ w3299]
          tunnel: w3278 -> [_ w3298]
          tunnel: [_ w3291] -> w3288
          tunnel: [_ w3290] -> w3287
          tunnel: [_ w3289] -> w3286
          frame False {
          }
          frame True {
            n2244 = local read "ValidationResults"() -> (w3295:waveform(dbl)[][])
            n2245 = local read "ValidationPos2"() -> (w3297:T3)
            n2246 = local read "ValidationPos1"() -> (w3296:T3)
            n2247 = Index Array(array=w3295, index (row)=w3298) -> (element=w3289:waveform(dbl)[])  [unwired: 1 in]
            n2248 = Index Array(array=w3296, index=w3298) -> (element=w3291:T9)
            n2249 = Index Array(array=w3297, index=w3298) -> (element=w3290:T9)
            n2250 = Index Array(array=w3289) -> (element=w3292:waveform(dbl))  [unwired: 1 in]
            n2251 = call "calculateJumperRiseAndFallTime-v03.vi"("jumptestMonitor"=w3292, "output cluster"=w3299) -> ("fall time (ms)"=w3293:dbl, "rise time (ms)"=w3294:dbl)  [unwired: 8 in]
            n2252 = local write "Validation Fall Time"(w3293) -> ()
            n2253 = local write "Validation Rise Time"(w3294) -> ()
          }
        }
      }
    }
    n2254 = local read "Save Resistance"() -> (w3141:bool)
    n2255 = case shown="False" w3141 {
      frame False {
        n2256 = local read "P1"() -> (w3147:dbl)
        n2257 = local write "Saved Pipette Resistance"(w3147) -> ()
      }
      frame True {
      }
    }
    n2258 = local read "stop always"() -> (w3144:bool)
    n2259 = local write "Wave Rise Time"(w3135) -> ()
    n2260 = local write "Jump Rise Time"(w3138) -> ()
    n2261 = local write "cells selected"(w3139) -> ()
    n2262 = local write "ValResult"(w3132) -> ()
    n2263 = local write "ValPos1"(w3133) -> ()
    n2264 = local write "Wave Fall Time"(w3136) -> ()
    n2265 = local write "Jump Fall Time"(w3137) -> ()
    n2266 = local write "ValPos2"(w3134) -> ()
    n2267 = local write "cells left"(w3140) -> ()
    n2268 = Wait (ms)(milliseconds to wait=u32 50) -> ()  [unwired: 1 out]
  }
  n2269 = Merge Errors(w400, w397) -> (w399:errorcluster)
  n2270 = Release Notifier(notifier=w401, error in (no error)=w399) -> ()  [unwired: 1 in, 3 out]
  n2271 = call "IMAQ Dispose"("All Images? (No)"=FALSE, "Image"=w677, "error in (no error)"=w676) -> ()  [unwired: 3 in, 1 out]
  n2272 = call "IMAQ Dispose"("All Images? (No)"=FALSE, "Image"=w680, "error in (no error)"=w681) -> ("error out"=w661:errorcluster)  [unwired: 3 in]
  n2273 = call "close_cam_topLvl_v02.vi"("error in (no error)"=w661, "cam info in"=w660) -> ()  [unwired: 9 in, 1 out]
